vi "Main.vi"() -> ()   [LabVIEW 2018]
doc: "This template is for the Queued Message Handler design pattern.\n\nThe Event Handling Loop generates messages based on user interface actions.\n\nThe Message Handling Loop processes messages generated by the Event Handling Loop, or by other messages. The messages are string values, so new messages can be added easily to the Message Cases case structure in the Message Handling Loop. Each message cluster can also provide an optional value for Message Data, which is a variant that can be converted to whatever message-specific data is required."
uses:
  controls/UI Data.ctl
  <vilib>/Utility/miscctls.llb/LVPointDoubleTypeDef.ctl
  <vilib>/Utility/miscctls.llb/LVPoint32TypeDef.ctl
  support/Message Queue/Enqueue Message (Single).vi
  <vilib>/Utility/error.llb/Error Cluster From Error Code.vi
  <vilib>/ErrorRing/Error Ring.xnode
  support/Message Queue/Message Queue.lvlib
  support/User Event - Stop/User Event - Stop.lvlib
  Manipulate IPF/Manipulate IPF.lvlib
panel:
  in  "Not Fitted Components":i32(listbox)
  in  "Not Tested Components":i32(listbox)
  in  "Enable Labels":bool caption="Labels"
  in  "Enable Not Fited Components":bool caption="Not Fited Components"
  in  "Enable Not Tested Components":bool caption="Not Tested Components"
  out "XY Graph":cluster{dbl[], dbl[]}[](graph)
  out "Event Log":string
  in  "Save  to file":bool
  in  "Reload":bool
  in  "Exit Button":bool
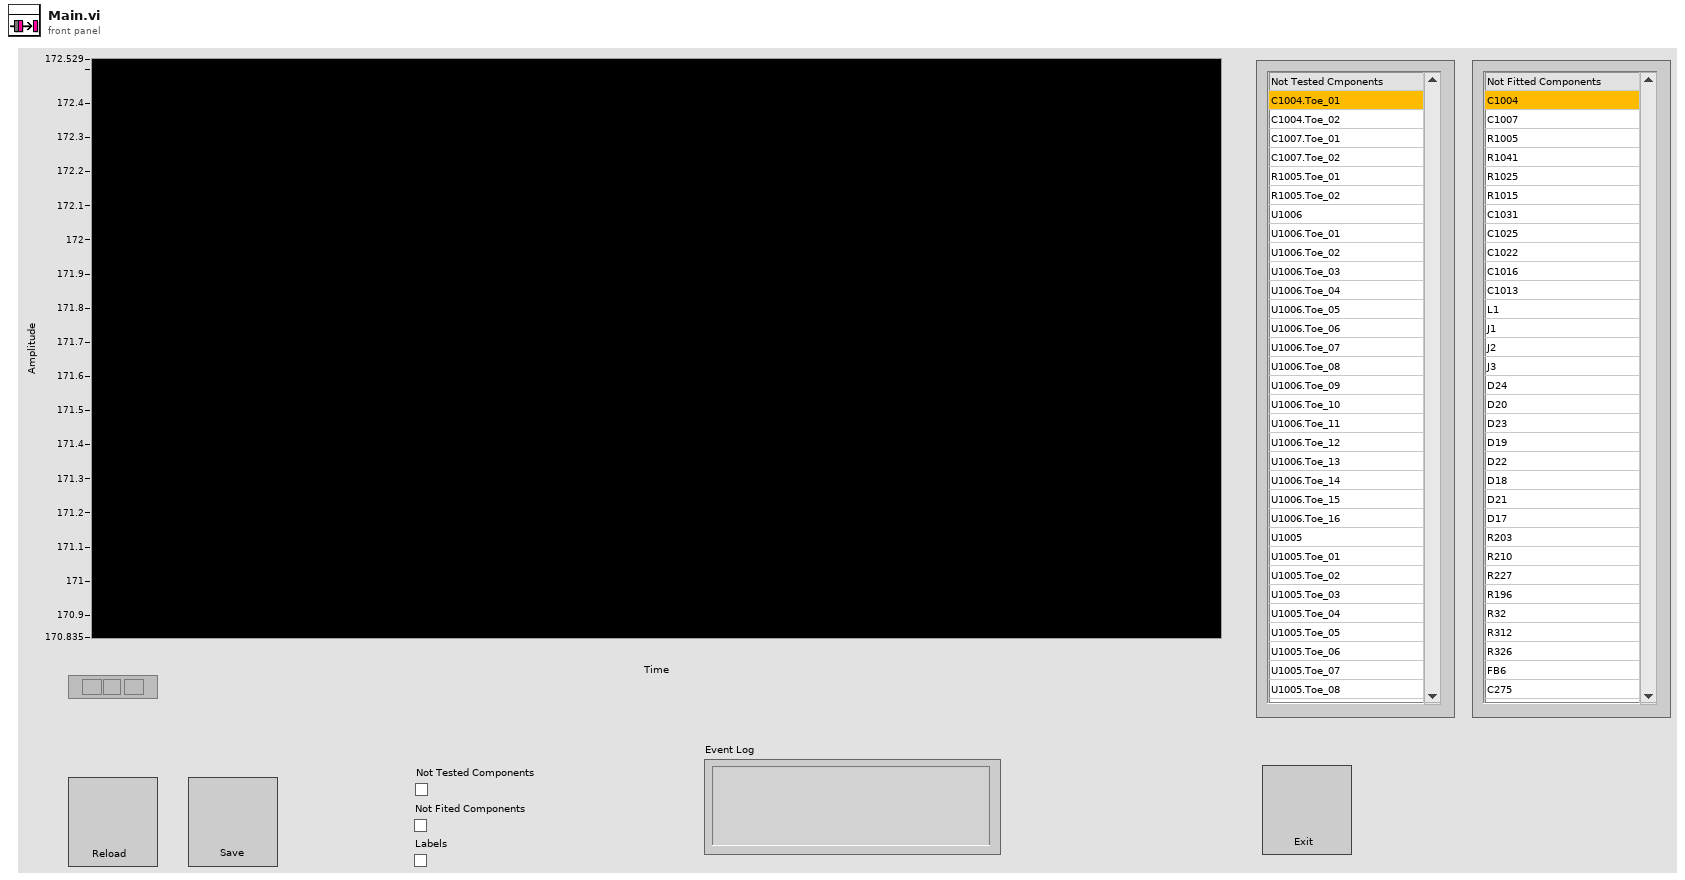
[diagram p1: front panel]
types:
  T1 = typedef "UI Data.ctl" = cluster{"Boolean <Replace Me>":bool, "String <Replace Me>":string, "Numeric <Replace Me>":dbl, "Do Something Ref":refnum<vi>, "Do Something Else Ref":refnum<vi>, "Data Display Ref":refnum<vi>, "Exit Button Ref":refnum<vi>, "CAD_Data":cluster{dbl[], dbl[]}[], "Reference":cluster{"XY Graph":refnum<vi>, "Not Tested Components":refnum<vi>, "Not Fitted Components":refnum<vi>, "Enable Not Fited Components":refnum<vi>, "Enable Not Tested Components":refnum<vi>, "Enable Labels":refnum<vi>}, "CAD data Origin":cluster{"Not fitted components":string[], "Not tested components":string[], "Not Fitted position[x][y] ":dbl[][], "Not Tested position[x][y]":dbl[][], "CAD Layers":cluster{"1st Filtered Array out":sgl[], "2nd Filtered Array out":sgl[]}[], "Xyz File Exist? ":bool, "Options":cluster{"Enable Not Tested Components":bool, "Enable Not Fited Components":bool, "Enable Labels":bool}, "Origin XY Scale Ranges":cluster{"XScale.Max":dbl, "XScale.Min":dbl, "YScale.Max":dbl, "YScale.Min":dbl}}, "CAD data Update":cluster{"Not fitted components":string[], "Not tested components":string[], "Not Fitted position[x][y] ":dbl[][], "Not Tested position[x][y]":dbl[][], "CAD Layers":cluster{"1st Filtered Array out":sgl[], "2nd Filtered Array out":sgl[]}[], "Xyz File Exist? ":bool, "Options":cluster{"Enable Not Tested Components":bool, "Enable Not Fited Components":bool, "Enable Labels":bool}, "Origin XY Scale Ranges":cluster{"XScale.Max":dbl, "XScale.Min":dbl, "YScale.Max":dbl, "YScale.Min":dbl}}}
  T2 = typedef "Message Queue.lvlib/All Message Queues.ctl" = cluster{"UI":refnum<queue>}
  T3 = typedef "LVPoint32TypeDef.ctl" = cluster{"Horizontal":i32, "Vertical":i32}
  T4 = cluster{"Enable Not Tested Components":bool, "Enable Not Fited Components":bool, "Enable Labels":bool}
  T5 = typedef "LVPointDoubleTypeDef.ctl" = cluster{"X":dbl, "Y":dbl}
  T6 = cluster{"Name":string, "Color":u32, "Style":u8, "Point Style":u8, "Name Visible":bool, "Allow Drag":bool, "Annotation Mode":u32, "Plot":i32, "Index":i32, "Position":cluster{"X":dbl, "Y":dbl}, "X Scale":u32, "Y Scale":u32, "Show Arrow":bool, "Lock Name":bool, "Plot Area":i32, "Label Offset":cluster{"X":dbl, "Y":dbl}}
  T7 = cluster{"Not fitted components":string[], "Not tested components":string[], "Not Fitted position[x][y] ":dbl[][], "Not Tested position[x][y]":dbl[][], "CAD Layers":cluster{"1st Filtered Array out":sgl[], "2nd Filtered Array out":sgl[]}[], "Xyz File Exist? ":bool, "Options":cluster{"Enable Not Tested Components":bool, "Enable Not Fited Components":bool, "Enable Labels":bool}, "Origin XY Scale Ranges":cluster{"XScale.Max":dbl, "XScale.Min":dbl, "YScale.Max":dbl, "YScale.Min":dbl}}
  T8 = cluster{"1st Filtered Array out":sgl[], "2nd Filtered Array out":sgl[]}[]
  T9 = cluster{"XScale.Max":dbl, "XScale.Min":dbl, "YScale.Max":dbl, "YScale.Min":dbl}
  T10 = cluster{"XScale.Offset":dbl, "YScale.Offset":dbl}
  T11 = cluster{"XScale.Multiplier":dbl, "YScale.Multiplier":dbl}
  T12 = cluster{"Name":string, "Color":u32, "Style":u8, "Point Style":u8, "Name Visible":bool, "Allow Drag":bool, "Annotation Mode":u32, "Plot":i32, "Index":i32, "Position":cluster{"X":dbl, "Y":dbl}, "X Scale":u32, "Y Scale":u32, "Show Arrow":bool, "Lock Name":bool, "Plot Area":i32, "Label Offset":cluster{"X":dbl, "Y":dbl}}[]
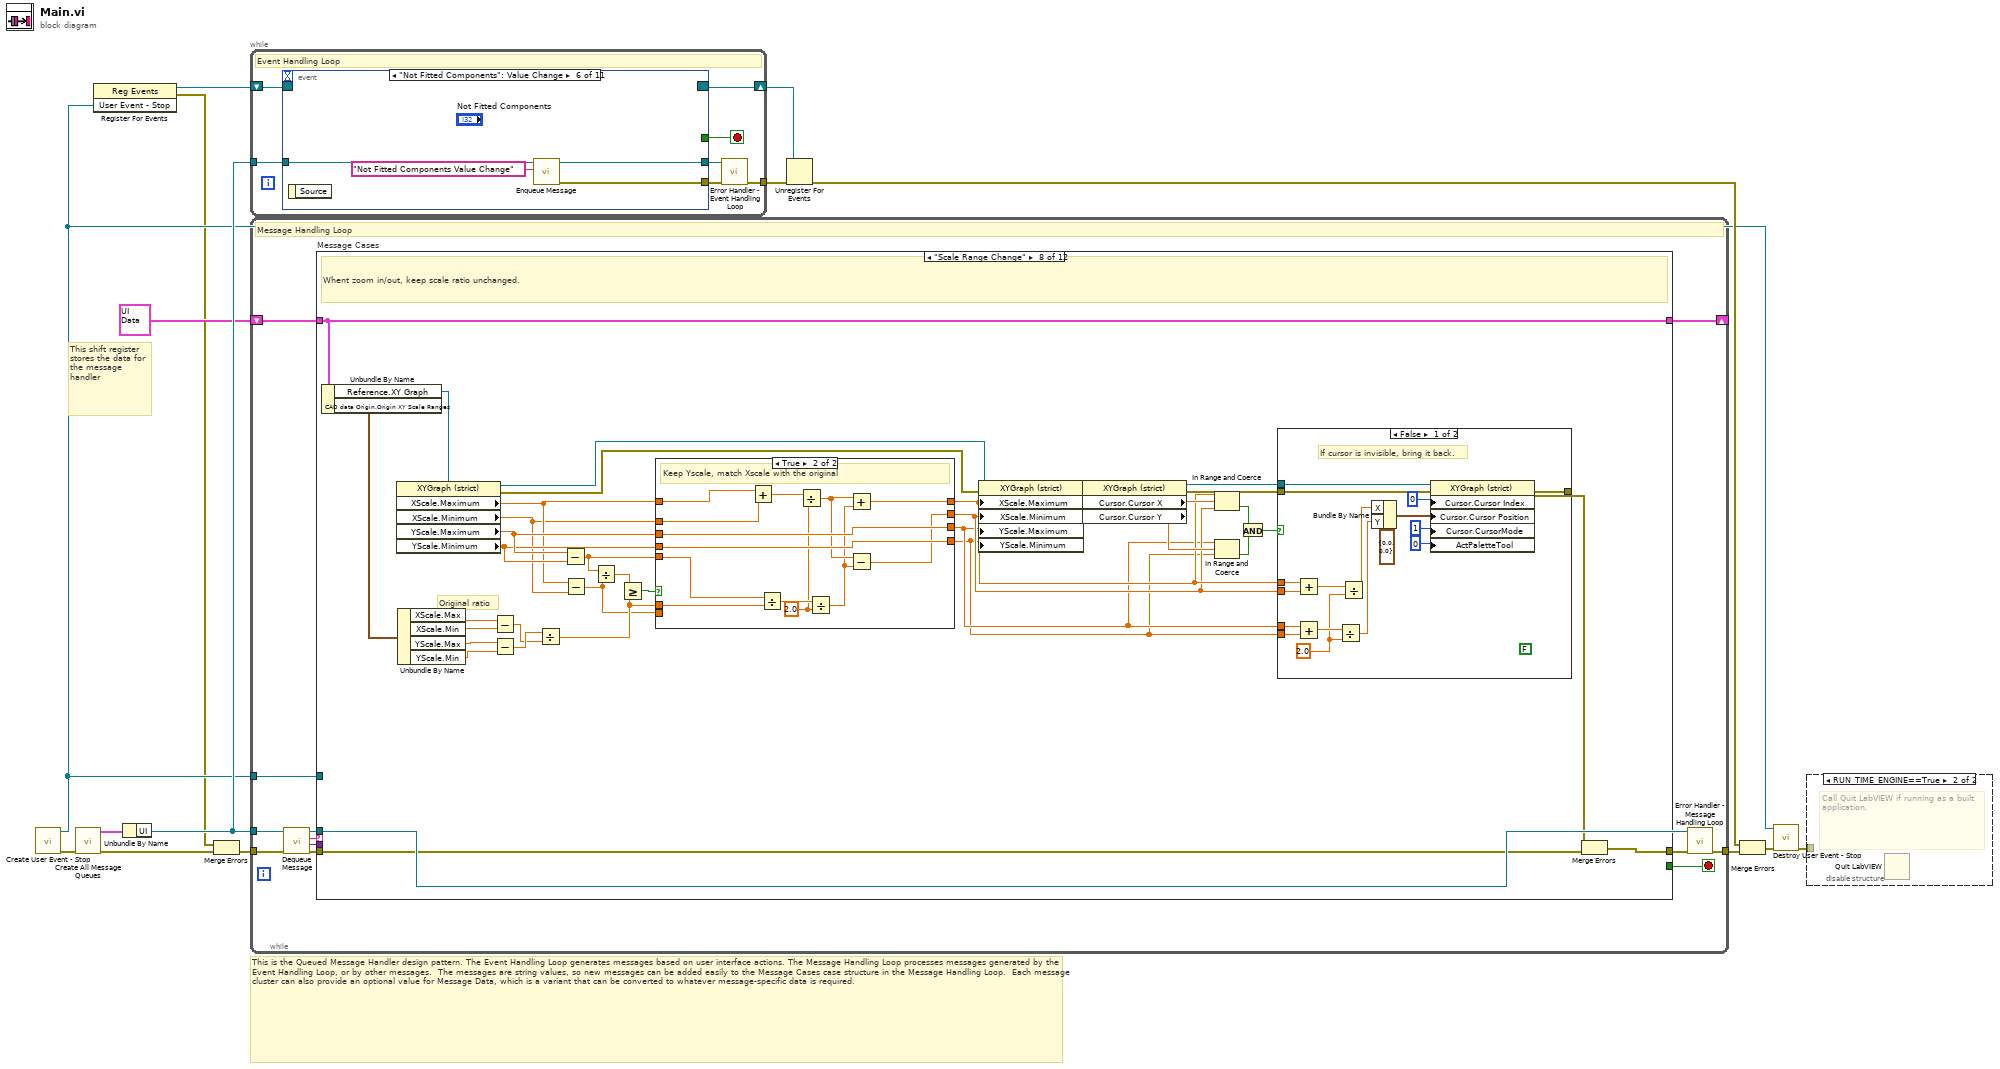
[diagram p0: block diagram]
diagram:
  # "This is the Queued Message Handler design pattern. The Event Handling Loop generates messages based on user interface actions. The Message Handling Loop processes messages generated by the Event Handling Loop, or by other messages.  The messages are string values, so new messages can be added easily to the Message Cases case structure in the Message Handling Loop.  Each message cluster can also provide an optional value for Message Data, which is a variant that can be converted to whatever message-specific data is required."
  # "This shift register stores the data for the message handler"
  n1 = call "Create User Event - Stop.vi"() -> ("error out"=w11:errorcluster, "User Event - Stop"=w3:refnum<user-event>)  [unwired: 10 in]
  n2 = call "Create All Message Queues.vi"("error in (no error)"=w11) -> ("error out"=w15:errorcluster, "Message Queues out"=w14:T2)  [unwired: 9 in]
  n3 = register-events(w3) -> (reference out=w4:refnum<event-registration>, error out=w1:errorcluster)  [unwired: 2 in]
  n4 = Unbundle By Name(w14) -> ("UI"=w12:refnum<queue>)
  n5 = Merge Errors(w1, w15) -> (w2:errorcluster)
  n6 = while {
    tunnel: w12 -> [w22]
    shift-right: [w20] -> w8
    shift-left: w4 -> [w21]
    tunnel: [w16] -> w5
    stop <- w18 stop-if-true
    # "Event Handling Loop"
    n7 = event shown="[5] \"Not Fitted Components\": Value Change" {
      selector: w21 -> [_ _ _ _ _ _ _ _ _ _ _]
      dyn-events: [_ _ _ _ _ _ _ _ _ _ _] -> w20
      timeout: _ -> [_ _ _ _ _ _ _ _ _ _ _]
      tunnel: [_ _ _ _ _ _ _ _ _ _ TRUE ("Discard?")] -> w18
      tunnel: w22 -> [w26 w30 w33 w37 w41 w45 w49 w54 w56 w61 w64]
      tunnel: [w23 _ _ w35 w38 w42 w46 w53 _ w60 _] -> w19
      tunnel: [w25 w29 w32 w36 w40 w44 w48 w52 w56 w59 w64] -> w17
      event "Reload": Value Change {
        # "#CodeNeeded - Send the appropriate message for this user interface event."
        n8 = event-data() -> ()  [unwired: 1 in, 1 out]
        n9 = call-poly "Enqueue Message.vi"("Message"="Reload", "Message Queue"=w26) -> ("error out"=w23:errorcluster, "dup Message Queue"=w25:refnum<queue>)  [unwired: 8 in]
      }
      event "XY Graph": Mouse Up {
        n10 = event-data() -> ("Coords"=w27:T3)  [unwired: 1 in]
        n11 = call-poly "Enqueue Message.vi"("Message Data"=w27, "Message"="Mouse Up", "Message Queue"=w30) -> ("dup Message Queue"=w29:refnum<queue>)  [unwired: 7 in, 1 out]
      }
      event "Enable Not Tested Components", "Enable Not Fited Components", "Enable Labels": Value Change {
        n12 = event-data() -> ()  [unwired: 1 in, 1 out]
        n13 = call-poly "Enqueue Message.vi"("Message"="Update CAD Layers", "Message Queue"=w33) -> ("dup Message Queue"=w32:refnum<queue>)  [unwired: 8 in, 1 out]
      }
      event "XY Graph": Scale Range Change {
        n14 = event-data() -> ()  [unwired: 1 in, 1 out]
        n15 = call-poly "Enqueue Message.vi"("Message"="Scale Range Change", "Message Queue"=w37) -> ("error out"=w35:errorcluster, "dup Message Queue"=w36:refnum<queue>)  [unwired: 8 in]
      }
      event "Not Tested Components": Value Change {
        n16 = event-data() -> ()  [unwired: 1 in, 1 out]
        n17 = call-poly "Enqueue Message.vi"("Message"="Not Fitted Components Value Change", "Message Queue"=w41) -> ("error out"=w38:errorcluster, "dup Message Queue"=w40:refnum<queue>)  [unwired: 8 in]
      }
      event "Not Fitted Components": Value Change {
        n18 = event-data() -> ()  [unwired: 1 in, 1 out]
        n19 = call-poly "Enqueue Message.vi"("Message"="Not Fitted Components Value Change", "Message Queue"=w45) -> ("error out"=w42:errorcluster, "dup Message Queue"=w44:refnum<queue>)  [unwired: 8 in]
      }
      event "Save  to file": Value Change {
        # "#CodeNeeded - Send the appropriate message for this user interface event."
        n20 = event-data() -> ()  [unwired: 1 in, 1 out]
        n21 = call-poly "Enqueue Message.vi"("Message"="Save to file", "Message Queue"=w49) -> ("error out"=w46:errorcluster, "dup Message Queue"=w48:refnum<queue>)  [unwired: 8 in]
      }
      event Panel Close? {
        # "Send the 'Confirm Quit' message if the user closes the panel of the VI. Discard the event so the 'Confirm Quit' message has a chance to run."
        n22 = event-data() -> ()  [unwired: 1 in, 1 out]
        n23 = call-poly "Enqueue Message.vi"("Priority Message? (F)"=TRUE, "Message"="Confirm Quit", "Message Queue"=w54) -> ("error out"=w53:errorcluster, "dup Message Queue"=w52:refnum<queue>)  [unwired: 7 in]
        n24 = event-data("Discard?"=TRUE) -> ()  [unwired: 1 in, 1 out]
      }
      event Application Instance Close {
        # "#CodeRecommended - When a project closes, all VIs within that project are aborted and leave memory. However, any code placed in this event frame is guaranteed to run to completion, so add any cleanup code that absolutely must happen here."
        n25 = event-data() -> ()  [unwired: 1 in, 1 out]
      }
      event "Exit Button": Value Change {
        n26 = event-data() -> ()  [unwired: 1 in, 1 out]
        n27 = call-poly "Enqueue Message.vi"("Priority Message? (F)"=TRUE, "Message"="Exit", "Message Queue"=w61) -> ("error out"=w60:errorcluster, "dup Message Queue"=w59:refnum<queue>)  [unwired: 7 in]
      }
      event User Event {
        # "The Message Handling Loop processed an \"Exit\" message, which fired this event to stop the Event Handling Loop."
        n28 = event-data() -> ()  [unwired: 1 in, 1 out]
        n29 = local write "Event Log"("\"Exit\" button pressed" ("VI Stopped")) -> ()
      }
    }
    n30 = call "Error Handler - Event Handling Loop.vi"("error in (no error)"=w19, "Message Queue"=w17) -> ("dup error in"=w16:errorcluster)  [unwired: 8 in, 1 out]
  }
  n31 = while {
    tunnel: w12 -> [w68]
    shift-right: [w75] -> _
    shift-left: T1 {"Boolean <Replace Me>"=FALSE, "String <Replace Me>"="", "Numeric <Replace Me>"=0.0, "Do Something Ref"=refnum, "Do Something Else Ref"=refnum, "Data Display Ref"=refnum, "Exit Button Ref"=refnum, "CAD_Data"=[{array[1801 elements], array[1801 elements]}, {array[46807 elements], array[46807 elements]}, {array[492003 elements], array[492003 elements]}, {array[314618 elements], array[314618 elements]}, {array[31626 elements], array[31626 elements]}, {array[569211 elements], array[569211 elements]}], "Reference"={"XY Graph"=refnum, "Not Tested Components"=refnum, "Not Fitted Components"=refnum, "Enable Not Fited Components"=refnum, "Enable Not Tested Components"=refnum, "Enable Labels"=refnum}, "CAD data Origin"={"Not fitted components"=[], "Not tested components"=[], "Not Fitted position[x][y] "=[], "Not Tested position[x][y]"=[], "CAD Layers"=[], "Xyz File Exist? "=FALSE, "Options"={"Enable Not Tested Components"=FALSE, "Enable Not Fited Components"=FALSE, "Enable Labels"=FALSE}, "Origin XY Scale Ranges"={"XScale.Max"=0.0, "XScale.Min"=0.0, "YScale.Max"=0.0, "YScale.Min"=0.0}}, "CAD data Update"={"Not fitted components"=[], "Not tested components"=[], "Not Fitted position[x][y] "=[], "Not Tested position[x][y]"=[], "CAD Layers"=[], "Xyz File Exist? "=FALSE, "Options"={"Enable Not Tested Components"=FALSE, "Enable Not Fited Components"=FALSE, "Enable Labels"=FALSE}, "Origin XY Scale Ranges"={"XScale.Max"=0.0, "XScale.Min"=0.0, "YScale.Max"=0.0, "YScale.Min"=0.0}}} ("Data Cluster") -> [w76]
    tunnel: w3 -> [w73]
    tunnel: w2 -> [w72]
    tunnel: [w66] -> w13
    stop <- w74 stop-if-true
    # "Message Handling Loop"
    n32 = call "Dequeue Message.vi"("error in (no error)"=w72, "Message Queue"=w68) -> ("error out"=w71:errorcluster, "Message Data"=w69:variant, "Message"=w70:string, "dup Message Queue"=w67:refnum<queue>)  [unwired: 6 in]
    n33 = case "Message Cases" shown="\"Scale Range Change\"" w70 {
      selector: w70 -> [_ _ _ _ _ _ _ _ _ _ _ w371]
      tunnel: w67 -> [w106 w119 w125 _ _ w146 _ _ _ _ w370 _]
      tunnel: w71 -> [w113 w121 w127 w134 w143 w150 w153 w189 w251 w321 w363 _]
      tunnel: [w85 w115 w128 w135 w137 w148 w151 w188 w267 w320 w366 w372] -> w65
      tunnel: w76 -> [w102 w122 w129 w136 w142 w149 w152 w156 w253 w319 w369 w373]
      tunnel: [w112 w122 w129 w136 w142 w149 w152 w156 w240 w319 w369 w373] -> w75
      tunnel: [_ _ _ _ _ _ _ _ _ _ TRUE _] -> w74
      tunnel: w69 -> [_ _ _ w133 w141 _ _ _ _ w318 w360 _]
      tunnel: w73 -> [_ _ _ _ _ _ _ _ _ _ w365 _]
      frame "Initialize" {
        w96 = T7 {"Not fitted components"=["C1004", "C1007", "R1005", "R1041", "R1025", "R1015", "C1031", "C1025", "C1022", "C1016", "C1013", "L1", "J1", "J2", "J3", "D24", "D20", "D23", "D19", "D22", "D18", "D21", "D17", "R203", "R210", "R227", "R196", "R32", "R312", "R326", "FB6", "C275", "R177", "R178", "R97", "R129", "R124", "R71", "R264", "R232", "R46", "R287", "R288", "CON2", "CON4", "CON1", "C196", "J4", "R252", "R182", "R310", "R311", "R328", "R75", "R102", "U11", "CON3", "R7", "R2", "R1", "R21", "R11", "R9", "R13", "R16", "R15", "R5", "R17", "R10", "BRK1", "BRK9", "BRK11", "BRK10", "BRK7", "BRK8", "BRK12", "BRK2", "BRK6", "R224", "R228", "R229"], "Not tested components"=["C1004.Toe_01", "C1004.Toe_02", "C1007.Toe_01", "C1007.Toe_02", "R1005.Toe_01", "R1005.Toe_02", "U1006", "U1006.Toe_01", "U1006.Toe_02", "U1006.Toe_03", "U1006.Toe_04", "U1006.Toe_05", "U1006.Toe_06", "U1006.Toe_07", "U1006.Toe_08", "U1006.Toe_09", "U1006.Toe_10", "U1006.Toe_11", "U1006.Toe_12", "U1006.Toe_13", "U1006.Toe_14", "U1006.Toe_15", "U1006.Toe_16", "U1005", "U1005.Toe_01", "U1005.Toe_02", "U1005.Toe_03", "U1005.Toe_04", "U1005.Toe_05", "U1005.Toe_06", "U1005.Toe_07", "U1005.Toe_08", "U1005.Toe_09", "U1005.Toe_10", "U1005.Toe_11", "U1005.Toe_12", "U1005.Toe_13", "U1005.Toe_14", "U1005.Toe_15", "U1005.Toe_16", "U1003", "U1003.Toe_01", "U1003.Toe_02", "U1003.Toe_03", "U1003.Toe_04", "U1003.Toe_05", "U1003.Toe_06", "U1003.Toe_07", "U1003.Toe_08", "U1003.Toe_09", "U1003.Toe_10", "U1003.Toe_11", "U1003.Toe_12", "U1003.Toe_13", "U1003.Toe_14", "U1003.Toe_15", "U1003.Toe_16", "U1003.Toe_17", "U1003.Toe_18", "U1003.Toe_19", "U1003.Toe_20", "U1003.Toe_21", "U1003.Toe_22", "U1003.Toe_23", "U1003.Toe_24", "U1003.Toe_25", "U1003.Toe_26", "U1003.Toe_27", "U1003.Toe_28", "U1003.Toe_29", "U1003.Toe_30", "U1003.Toe_31", "U1003.Toe_32", "U1003.Toe_33", "U1003.Toe_34", "U1003.Toe_35", "U1003.Toe_36", "U1003.Toe_37", "U1003.Toe_38", "U1002", "U1002.Toe_01", "U1002.Toe_02", "U1002.Toe_03", "U1002.Toe_04", "U1002.Toe_05", "U1002.Toe_06", "U1002.Toe_07", "U1002.Toe_08", "U1002.Toe_09", "U1002.Toe_10", "U1002.Toe_11", "U1002.Toe_12", "U1002.Toe_13", "U1002.Toe_14", "U1002.Toe_15", "U1002.Toe_16", "U1002.Toe_17", "U1002.Toe_18", "U1002.Toe_19", "U1002.Toe_20", "U1002.Toe_21", "U1002.Toe_22", "U1002.Toe_23", "U1002.Toe_24", "U1002.Toe_25", "U1002.Toe_26", "U1002.Toe_27", "U1002.Toe_28", "U1002.Toe_29", "U1002.Toe_30", "U1002.Toe_31", "U1002.Toe_32", "U1002.Toe_33", "U1002.Toe_34", "U1002.Toe_35", "U1002.Toe_36", "U1002.Toe_37", "U1002.Toe_38", "U1001", "U1001.Toe_01", "U1001.Toe_02", "U1001.Toe_03", "U1001.Toe_04", "U1001.Toe_05", "U1001.Toe_06", "U1001.Toe_07", "U1001.Toe_08", "U1001.Toe_09", "U1001.Toe_10", "U1001.Toe_11", "U1001.Toe_12", "U1001.Toe_13", "U1001.Toe_14", "U1001.Toe_15", "U1001.Toe_16", "U1001.Toe_17", "U1001.Toe_18", "U1001.Toe_19", "U1001.Toe_20", "U1001.Toe_21", "U1001.Toe_22", "U1001.Toe_23", "U1001.Toe_24", "U1001.Toe_25", "U1001.Toe_26", "U1001.Toe_27", "U1001.Toe_28", "U1001.Toe_29", "U1001.Toe_30", "U1001.Toe_31", "U1001.Toe_32", "U1001.Toe_33", "U1001.Toe_34", "U1001.Toe_35", "U1001.Toe_36", "U1001.Toe_37", "U1001.Toe_38", "U1000", "U1000.Toe_01", "U1000.Toe_02", "U1000.Toe_03", "U1000.Toe_04", "U1000.Toe_05", "U1000.Toe_06", "U1000.Toe_07", "U1000.Toe_08", "U1000.Toe_09", "U1000.Toe_10", "U1000.Toe_11", "U1000.Toe_12", "U1000.Toe_13", "U1000.Toe_14", "U1000.Toe_15", "U1000.Toe_16", "U1000.Toe_17", "U1000.Toe_18", "U1000.Toe_19", "U1000.Toe_20", "U1000.Toe_21", "U1000.Toe_22", "U1000.Toe_23", "U1000.Toe_24", "U1000.Toe_25", "U1000.Toe_26", "U1000.Toe_27", "U1000.Toe_28", "U1000.Toe_29", "U1000.Toe_30", "U1000.Toe_31", "U1000.Toe_32", "U1000.Toe_33", "U1000.Toe_34", "U1000.Toe_35", "U1000.Toe_36", "U1000.Toe_37", "U1000.Toe_38", "R1041.Toe_01", "R1041.Toe_02", "R1025.Toe_01", "R1025.Toe_02", "R1015.Toe_01", "R1015.Toe_02", "C1031.Toe_01", "C1031.Toe_02", "C1025.Toe_01", "C1025.Toe_02", "C1022.Toe_01", "C1022.Toe_02", "C1016.Toe_01", "C1016.Toe_02", "C1013.Toe_01", "C1013.Toe_02", "L1.Toe_01", "L1.Toe_02", "L1.Toe_NPTH", "L1.Toe_NPTH", "L1.Toe_NPTH", "L1.Toe_NPTH", "J1", "J1.Toe_01", "J1.Toe_02", "J1.Toe_03", "J2", "J2.Toe_01", "J2.Toe_02", "J2.Toe_03", "J3", "J3.Toe_01", "J3.Toe_02", "J3.Toe_03", "U9", "U9.Toe_01", "U9.Toe_02", "U9.Toe_03", "U9.Toe_04", "U9.Toe_05", "U9.Toe_09", "U9.Toe_10", "U9.Toe_11", "U9.Toe_12", "U9.Toe_13", "U9.Toe_14", "U9.Toe_15", "L2", "L2.Toe_01", "L2.Toe_02", "D6", "D6.Toe_0A", "D6.Toe_0C", "D7", "D7.Toe_0A", "D7.Toe_0C", "D8", "D8.Toe_0A", "D8.Toe_0C", "D5", "D5.Toe_0A", "D5.Toe_0C", "U15", "U15.Toe_02", "U15.Toe_03", "U15.Toe_04", "U15.Toe_08", "D24.Toe_0A", "D24.Toe_0C", "D20", "D20.Toe_0A", "D20.Toe_0C", "D23.Toe_0A", "D23.Toe_0C", "D19", "D19.Toe_0A", "D19.Toe_0C", "D22.Toe_0A", "D22.Toe_0C", "D18", "D18.Toe_0A", "D18.Toe_0C", "D21.Toe_0A", "D21.Toe_0C", "D17", "D17.Toe_0A", "D17.Toe_0C", "D16", "D16.Toe_0A", "D16.Toe_0C", "D12", "D12.Toe_0A", "D12.Toe_0C", "D15", "D15.Toe_0A", "D15.Toe_0C", "D11", "D11.Toe_0A", "D11.Toe_0C", "D14", "D14.Toe_0A", "D14.Toe_0C", "D10", "D10.Toe_0A", "D10.Toe_0C", "D9", "D9.Toe_0A", "D9.Toe_0C", "D13", "D13.Toe_0A", "D13.Toe_0C", "Q19", "Q19.Toe_01", "Q19.Toe_02", "Q19.Toe_03", "Q23", "Q23.Toe_01", "Q23.Toe_02", "Q23.Toe_03", "Q23.Toe_04", "Q23.Toe_06", "Q23.Toe_07", "Q23.Toe_08", "Q20", "Q20.Toe_01", "Q20.Toe_02", "Q20.Toe_03", "Q24", "Q24.Toe_01", "Q24.Toe_02", "Q24.Toe_03", "Q24.Toe_04", "Q24.Toe_06", "Q24.Toe_07", "Q24.Toe_08", "Q21", "Q21.Toe_01", "Q21.Toe_02", "Q21.Toe_03", "R203.Toe_01", "R203.Toe_02", "R210.Toe_01", "R210.Toe_02", "U24", "U24.Toe_01", "U24.Toe_02", "U24.Toe_03", "U24.Toe_04", "U24.Toe_05", "U24.Toe_06", "U24.Toe_07", "U24.Toe_08", "U19", "U19.Toe_01", "U19.Toe_02", "U19.Toe_03", "U19.Toe_04", "U19.Toe_05", "U19.Toe_06", "U19.Toe_07", "U19.Toe_08", "U19.Toe_09", "U19.Toe_10", "U19.Toe_11", "U19.Toe_12", "U19.Toe_13", "U19.Toe_14", "U19.Toe_15", "U19.Toe_16", "U25", "U25.Toe_01", "U25.Toe_02", "U25.Toe_03", "U25.Toe_04", "U25.Toe_05", "U25.Toe_06", "U25.Toe_07", "U25.Toe_08", "U20", "U20.Toe_01", "U20.Toe_02", "U20.Toe_03", "U20.Toe_04", "U20.Toe_05", "U20.Toe_06", "U20.Toe_07", "U20.Toe_08", "U20.Toe_09", "U20.Toe_10", "U20.Toe_11", "U20.Toe_12", "U20.Toe_13", "U20.Toe_14", "U20.Toe_15", "U20.Toe_16", "U16", "U16.Toe_02", "U16.Toe_03", "U16.Toe_04", "U16.Toe_08", "U26", "U26.Toe_01", "U26.Toe_02", "U26.Toe_03", "U26.Toe_04", "U26.Toe_05", "U26.Toe_06", "U26.Toe_07", "U26.Toe_08", "U21", "U21.Toe_01", "U21.Toe_02", "U21.Toe_03", "U21.Toe_04", "U21.Toe_05", "U21.Toe_06", "U21.Toe_07", "U21.Toe_08", "U21.Toe_09", "U21.Toe_10", "U21.Toe_11", "U21.Toe_12", "U21.Toe_13", "U21.Toe_14", "U21.Toe_15", "U21.Toe_16", "U17", "U17.Toe_02", "U17.Toe_03", "U17.Toe_04", "U17.Toe_08", "Q18", "Q18.Toe_01", "Q18.Toe_02", "Q18.Toe_03", "Q22", "Q22.Toe_01", "Q22.Toe_02", "Q22.Toe_03", "Q22.Toe_04", "Q22.Toe_06", "Q22.Toe_07", "Q22.Toe_08", "R227.Toe_01", "R227.Toe_02", "R196.Toe_01", "R196.Toe_02", "U23", "U23.Toe_01", "U23.Toe_02", "U23.Toe_03", "U23.Toe_04", "U23.Toe_05", "U23.Toe_06", "U23.Toe_07", "U23.Toe_08", "U18", "U18.Toe_01", "U18.Toe_02", "U18.Toe_03", "U18.Toe_04", "U18.Toe_05", "U18.Toe_06", "U18.Toe_07", "U18.Toe_08", "U18.Toe_09", "U18.Toe_10", "U18.Toe_11", "U18.Toe_12", "U18.Toe_13", "U18.Toe_14", "U18.Toe_15", "U18.Toe_16", "U14", "U14.Toe_02", "U14.Toe_03", "U14.Toe_04", "U14.Toe_08", "U27", "U27.Toe_01", "U27.Toe_02", "U27.Toe_03", "Q6", "Q6.Toe_01", "Q6.Toe_02", "Q6.Toe_03", "U2", "U2.Toe_01", "U2.Toe_02", "U2.Toe_03", "U2.Toe_04", "U2.Toe_05", "U2.Toe_06", "U2.Toe_07", "U2.Toe_08", "U2.Toe_09", "U2.Toe_10", "U2.Toe_11", "U2.Toe_12", "U2.Toe_13", "U2.Toe_14", "U2.Toe_15", "U2.Toe_16", "U2.Toe_17", "U2.Toe_18", "U2.Toe_19", "U2.Toe_20", "U2.Toe_21", "U2.Toe_22", "U2.Toe_23", "U2.Toe_24", "U2.Toe_25", "U2.Toe_26", "U2.Toe_27", "U2.Toe_28", "U2.Toe_29", "U2.Toe_30", "U2.Toe_31", "U2.Toe_32", "U2.Toe_33", "U2.Toe_34", "U2.Toe_35", "U2.Toe_36", "U2.Toe_37", "U2.Toe_38", "U2.Toe_39", "U2.Toe_40", "U2.Toe_41", "U2.Toe_42", "U2.Toe_43", "U2.Toe_44", "U2.Toe_45", "U2.Toe_46", "U2.Toe_47", "U2.Toe_48", "U2.Toe_49", "U2.Toe_50", "U2.Toe_51", "U2.Toe_52", "U2.Toe_53", "U2.Toe_54", "R32.Toe_01", "R32.Toe_02", "Q7", "Q7.Toe_01", "Q7.Toe_02", "Q7.Toe_03", "Q8", "Q8.Toe_01", "Q8.Toe_02", "Q8.Toe_03", "FB1", "FB1.Toe_01", "FB1.Toe_02", "Q17", "Q17.Toe_01", "Q17.Toe_02", "Q17.Toe_03", "Q14", "Q14.Toe_01", "Q14.Toe_02", "Q14.Toe_03", "Q11", "Q11.Toe_01", "Q11.Toe_02", "Q11.Toe_03", "R312.Toe_01", "R312.Toe_02", "R326.Toe_01", "R326.Toe_02", "L3", "L3.Toe_01", "L3.Toe_02", "L3.Toe_03", "L3.Toe_04", "FB6.Toe_01", "FB6.Toe_02", "FB7", "FB7.Toe_01", "FB7.Toe_02", "C275.Toe_01", "C275.Toe_02", "R177.Toe_01", "R177.Toe_02", "R178.Toe_01", "R178.Toe_02", "U36", "U36.Toe_01", "U36.Toe_02", "U36.Toe_03", "U36.Toe_04", "U36.Toe_05", "U36.Toe_06", "U36.Toe_07", "U36.Toe_08", "U36.Toe_09", "U36.Toe_10", "U36.Toe_11", "U36.Toe_12", "U36.Toe_13", "U36.Toe_14", "U36.Toe_15", "U36.Toe_16", "U36.Toe_17", "U36.Toe_18", "U36.Toe_19", "U36.Toe_20", "U36.Toe_21", "U36.Toe_22", "U36.Toe_23", "U36.Toe_24", "U36.Toe_25", "U36.Toe_26", "U36.Toe_27", "U36.Toe_28", "U36.Toe_29", "U36.Toe_30", "U36.Toe_31", "U36.Toe_32", "Q30", "Q30.Toe_01", "Q30.Toe_02", "Q30.Toe_03", "Q26", "Q26.Toe_01", "Q26.Toe_02", "Q26.Toe_03", "LED1", "LED1.Toe_01", "LED1.Toe_02", "LED1.Toe_03", "LED5", "LED5.Toe_01", "LED5.Toe_02", "LED5.Toe_03", "LED5.Toe_04", "U8", "U8.Toe_01", "U8.Toe_02", "U8.Toe_03", "U8.Toe_04", "U8.Toe_05", "U8.Toe_06", "U8.Toe_07", "U8.Toe_08", "U8.Toe_09", "U8.Toe_10", "U8.Toe_11", "U8.Toe_12", "U8.Toe_13", "U8.Toe_14", "U8.Toe_15", "U8.Toe_16", "U8.Toe_17", "U8.Toe_18", "U8.Toe_19", "U8.Toe_20", "U8.Toe_21", "U8.Toe_22", "U8.Toe_23", "U8.Toe_24", "U8.Toe_25", "U8.Toe_26", "U8.Toe_27", "U8.Toe_28", "U8.Toe_29", "U8.Toe_30", "U8.Toe_31", "U8.Toe_32", "U8.Toe_33", "U8.Toe_34", "U8.Toe_35", "U8.Toe_36", "U8.Toe_37", "U8.Toe_38", "U8.Toe_39", "U8.Toe_40", "U8.Toe_41", "U8.Toe_42", "U8.Toe_43", "U8.Toe_44", "U8.Toe_45", "U8.Toe_46", "U8.Toe_47", "U8.Toe_48", "U8.Toe_49", "U8.Toe_50", "U8.Toe_51", "U8.Toe_52", "U8.Toe_53", "U8.Toe_54", "U5", "U5.Toe_01", "U5.Toe_02", "U5.Toe_03", "U5.Toe_04", "U5.Toe_05", "U5.Toe_06", "U5.Toe_07", "U5.Toe_08", "U5.Toe_09", "U5.Toe_10", "U5.Toe_11", "U5.Toe_12", "U5.Toe_13", "U5.Toe_14", "U5.Toe_15", "U5.Toe_16", "U5.Toe_17", "U5.Toe_18", "U5.Toe_19", "U5.Toe_20", "U5.Toe_21", "U5.Toe_22", "U5.Toe_23", "U5.Toe_24", "U5.Toe_25", "U5.Toe_26", "U5.Toe_27", "U5.Toe_28", "U5.Toe_29", "U5.Toe_30", "U5.Toe_31", "U5.Toe_32", "U5.Toe_33", "U5.Toe_34", "U5.Toe_35", "U5.Toe_36", "U5.Toe_37", "U5.Toe_38", "U5.Toe_39", "U5.Toe_40", "U5.Toe_41", "U5.Toe_42", "U5.Toe_43", "U5.Toe_44", "U5.Toe_45", "U5.Toe_46", "U5.Toe_47", "U5.Toe_48", "U5.Toe_49", "U5.Toe_50", "U5.Toe_51", "U5.Toe_52", "U5.Toe_53", "U5.Toe_54", "U4", "U4.Toe_01", "U4.Toe_02", "U4.Toe_03", "U4.Toe_04", "U4.Toe_05", "U4.Toe_06", "U4.Toe_07", "U4.Toe_08", "U4.Toe_09", "U4.Toe_10", "U4.Toe_11", "U4.Toe_12", "U4.Toe_13", "U4.Toe_14", "U4.Toe_15", "U4.Toe_16", "U4.Toe_17", "U4.Toe_18", "U4.Toe_19", "U4.Toe_20", "U4.Toe_21", "U4.Toe_22", "U4.Toe_23", "U4.Toe_24", "U4.Toe_25", "U4.Toe_26", "U4.Toe_27", "U4.Toe_28", "U4.Toe_29", "U4.Toe_30", "U4.Toe_31", "U4.Toe_32", "U4.Toe_33", "U4.Toe_34", "U4.Toe_35", "U4.Toe_36", "U4.Toe_37", "U4.Toe_38", "U4.Toe_39", "U4.Toe_40", "U4.Toe_41", "U4.Toe_42", "U4.Toe_43", "U4.Toe_44", "U4.Toe_45", "U4.Toe_46", "U4.Toe_47", "U4.Toe_48", "U4.Toe_49", "U4.Toe_50", "U4.Toe_51", "U4.Toe_52", "U4.Toe_53", "U4.Toe_54", "R97.Toe_01", "R97.Toe_02", "R129.Toe_01", "R129.Toe_02", "R124.Toe_01", "R124.Toe_02", "R71.Toe_01", "R71.Toe_02", "R264.Toe_01", "R264.Toe_02", "R232.Toe_01", "R232.Toe_02", "R46.Toe_01", "R46.Toe_02", "R287.Toe_01", "R287.Toe_02", "R288.Toe_01", "R288.Toe_02", "Q33", "Q33.Toe_01", "Q33.Toe_02", "Q33.Toe_03", "Q32", "Q32.Toe_01", "Q32.Toe_02", "Q32.Toe_03", "Q16", "Q16.Toe_01", "Q16.Toe_02", "Q16.Toe_03", "Q15", "Q15.Toe_01", "Q15.Toe_02", "Q15.Toe_03", "Q31", "Q31.Toe_01", "Q31.Toe_02", "Q31.Toe_03", "Q29", "Q29.Toe_01", "Q29.Toe_02", "Q29.Toe_03", "Q13", "Q13.Toe_01", "Q13.Toe_02", "Q13.Toe_03", "Q12", "Q12.Toe_01", "Q12.Toe_02", "Q12.Toe_03", "Q28", "Q28.Toe_01", "Q28.Toe_02", "Q28.Toe_03", "Q27", "Q27.Toe_01", "Q27.Toe_02", "Q27.Toe_03", "Q10", "Q10.Toe_01", "Q10.Toe_02", "Q10.Toe_03", "Q9", "Q9.Toe_01", "Q9.Toe_02", "Q9.Toe_03", "LED4", "LED4.Toe_01", "LED4.Toe_02", "LED4.Toe_03", "LED8", "LED8.Toe_01", "LED8.Toe_02", "LED8.Toe_03", "LED8.Toe_04", "LED3", "LED3.Toe_01", "LED3.Toe_02", "LED3.Toe_03", "LED7", "LED7.Toe_01", "LED7.Toe_02", "LED7.Toe_03", "LED7.Toe_04", "LED2", "LED2.Toe_01", "LED2.Toe_02", "LED2.Toe_03", "LED6", "LED6.Toe_01", "LED6.Toe_02", "LED6.Toe_03", "LED6.Toe_04", "FB4", "FB4.Toe_01", "FB4.Toe_02", "FB3", "FB3.Toe_01", "FB3.Toe_02", "FB2", "FB2.Toe_01", "FB2.Toe_02", "CON2.Toe_A1", "CON2.Toe_A2", "CON2.Toe_A3", "CON2.Toe_A4", "CON2.Toe_A5", "CON2.Toe_A6", "CON2.Toe_A7", "CON2.Toe_A8", "CON2.Toe_A9", "CON2.Toe_A10", "CON2.Toe_B1", "CON2.Toe_B2", "CON2.Toe_B3", "CON2.Toe_B4", "CON2.Toe_B5", "CON2.Toe_B6", "CON2.Toe_B7", "CON2.Toe_B8", "CON2.Toe_B9", "CON2.Toe_B10", "CON2.Toe_C1", "CON2.Toe_C2", "CON2.Toe_C3", "CON2.Toe_C4", "CON2.Toe_C5", "CON2.Toe_C6", "CON2.Toe_C7", "CON2.Toe_C8", "CON2.Toe_C9", "CON2.Toe_C10", "CON2.Toe_D1", "CON2.Toe_D2", "CON2.Toe_D3", "CON2.Toe_D4", "CON2.Toe_D5", "CON2.Toe_D6", "CON2.Toe_D7", "CON2.Toe_D8", "CON2.Toe_D9", "CON2.Toe_D10", "CON2.Toe_E1", 